vi "SCAPE-SpatialResolutionNumericalSimulation-4.vi"() -> ()   [LabVIEW 2024]
uses:
  <vilib>/Analysis/coordinate.llb/3D Cartesian Coordinate Rotation (Euler) (Scalar).vi
  <vilib>/Analysis/_algsub.llb/Real Vector Norm.vi
  <vilib>/Analysis/NI_AALPro.lvlib
  <vilib>/vision/NI_Vision_Development_Module.lvlib
panel:
  in  "r increment":dbl=2.0
  out "index":i32
  in  "iterataion":i32=1
  out "Array 2":dbl[][](array[numeric])=[[0.297159721790366, 0.6131743105327635, 1.1542088695697097]]
  out "x*y":dbl=2.94
  out "PSFxy":u16[][](graph)
  out "PSFxz":u16[][](graph)
  in  "y":dbl=0.7
  out "Image 3":T1(plugin-control)
  out "Image":T1(plugin-control)
  out "xy":u16[][](graph)
  out "zx":u16[][](graph)
  out "size(s) 3":i32[](array[numeric])=[256, 335, 256]
  out "size(s) 2":i32[](array[numeric])=[335, 256, 256]
  out "size(s)":i32[](array[numeric])=[110, 256, 256]
  in  "Angle (degrees)":dbl=45.0 format="%.2f"
  in  "perpendicular(T)/parallel(F)":bool=TRUE
  out "element":i32=127
  out "FWHMz":dbl=1.1542088695697097
  out "PSFz":u16[](graph)=[402, 405, 408, 411, 413, 415, 416, 417, 419, 420, 422, 424, 426, 429, 433, 437, 443, 450, 459, 468, 479, 493, 507, 524, 542, 563, 585, 610, 637, 666, 696, 730, 765, 802, 842, 883, 926, 970, 1017, 1065, 1114, 1164, 1215, 1267, 1320, 1372, 1423, 1475, 1528, 1579, 1629, 1677, 1725, 1771, 1814, 1855, 1895, 1933, 1966, 1997, 2026, 2054, 2076, 2095, 2114, 2127, 2139, 2149, 2155, 2161, 2165, 2167, 2169, 2171, 2174, 2177, 2181, 2189, 2199, 2215, 2236, 2260, 2296, 2339, 2389, 2450, 2526, 2613, 2710, 2831, 2966, 3116, 3289, 3485, 3699, 3935, 4205, 4496, 4807, 5160, 5541, 5947, 6384, 6863, 7372, 7909, 8493, 9109, 9760, 10451, 11182, 11941, 12740, 13591, 14473, 15375, 16329, 17325, 18356, 19398, 20489, 21616, 22778, 23953, 25153, 26390, 27662, 28941, 30221, 31535, 32879, 34233, 35557, 36903, 38273, 39669, 40991, 42317, 43664, 45034, 46319, 47585, 48860, 50137, 51344, 52506, 53661, 54778, 55867, 56881, 57839, 58771, 59697, 60509, 61237, 61944, 62648, 63212, 63707, 64160, 64583, 64893, 65139, 65318, 65421, 65478, 65463, 65328, 65141, 64938, 64646, 64221, 63759, 63289, 62709, 62051, 61334, 60597, 59778, 58919, 57976, 56989, 55982, 54953, 53810, 52645, 51486, 50309, 49035, 47748, 46476, 45186, 43856, 42496, 41153, 39811, 38472, 37087, 35723, 34386, 33076, 31715, 30387, 29093, 27832, 26560, 25311, 24097, 22924, 21771, 20633, 19529, 18480, 17459, 16452, 15494, 14580, 13703, 12846, 12040, 11270, 10536, 9845, 9188, 8562, 7980, 7437, 6921, 6434, 5997, 5586, 5199, 4848, 4529, 4234, 3962, 3724, 3504, 3305, 3133, 2979, 2840, 2720, 2620, 2531, 2452, 2391, 2339, 2295, 2260, 2233, 2211, 2195, 2185, 2177, 2171, 2168, 2166, 2164, 2162, 2160, 2157, 2152, 2144, 2135, 2125, 2110, 2092, 2073, 2053, 2026, 1996, 1966, 1933, 1896, 1856, 1815, 1772, 1727, 1680, 1631, 1581, 1531, 1479, 1427, 1374, 1324, 1271, 1219, 1168, 1117, 1069, 1021, 974, 929, 886, 845, 805, 768, 733, 699, 668, 638, 611, 587, 565, 543, 525, 509, 494, 481, 470, 460, 452, 445, 439, 434, 430, 427, 425, 424, 423, 423, 422, 421, 421, 420, 418, 416, 414, 412, 408, 404, 400, 394]
  in  "astigmatism (lambda)":dbl
  out "sum 2":dbl=26023.862010898454
  in  "image scan":bool=TRUE
  out "PSFy":u16[](graph)=[27, 29, 30, 31, 32, 34, 36, 38, 40, 42, 43, 45, 47, 49, 50, 52, 53, 54, 55, 55, 56, 56, 56, 57, 57, 57, 58, 59, 60, 62, 64, 67, 70, 75, 79, 85, 90, 96, 103, 110, 118, 126, 133, 141, 149, 157, 164, 172, 179, 186, 193, 200, 207, 214, 222, 230, 239, 249, 260, 272, 286, 301, 317, 334, 353, 372, 393, 414, 437, 459, 482, 505, 530, 555, 582, 611, 643, 679, 724, 778, 842, 919, 1023, 1150, 1298, 1484, 1714, 1993, 2323, 2712, 3166, 3708, 4340, 5047, 5837, 6774, 7815, 8952, 10197, 11603, 13125, 14754, 16516, 18402, 20401, 22510, 24722, 27017, 29388, 31833, 34323, 36849, 39374, 41890, 44389, 46860, 49225, 51501, 53677, 55731, 57617, 59333, 60845, 62163, 63287, 64182, 64762, 65141, 65324, 65206, 64801, 64179, 63367, 62266, 60951, 59430, 57726, 55852, 53833, 51644, 49349, 46980, 44547, 42027, 39492, 36956, 34429, 31931, 29480, 27085, 24774, 22555, 20437, 18426, 16528, 14742, 13104, 11595, 10191, 8891, 7768, 6749, 5822, 4993, 4295, 3684, 3145, 2686, 2301, 1982, 1716, 1493, 1308, 1165, 1052, 958, 880, 823, 776, 736, 702, 673, 645, 620, 594, 569, 545, 519, 494, 469, 444, 419, 395, 372, 350, 330, 311, 293, 277, 263, 249, 238, 227, 216, 208, 199, 191, 183, 175, 167, 160, 152, 145, 137, 130, 122, 115, 108, 101, 95, 89, 83, 78, 74, 70, 67, 65, 63, 61, 59, 59, 58, 58, 58, 57, 57, 57, 57, 56, 55, 54, 53, 52, 50, 49, 46, 44, 42, 40, 38, 36, 35, 33, 30, 29, 28]
  out "PSFx":u16[](graph)=[0, 0, 0, 1, 3, 4, 6, 8, 9, 10, 10, 10, 9, 7, 5, 3, 2, 1, 0, 0, 2, 4, 7, 10, 13, 16, 18, 19, 19, 17, 15, 12, 8, 5, 2, 0, 0, 2, 5, 10, 16, 22, 28, 33, 36, 37, 35, 32, 26, 19, 12, 6, 2, 1, 3, 9, 18, 30, 45, 59, 72, 82, 88, 88, 83, 72, 58, 41, 25, 11, 3, 3, 13, 32, 61, 98, 139, 180, 218, 248, 264, 266, 250, 219, 175, 125, 75, 36, 15, 22, 64, 144, 263, 417, 597, 790, 979, 1150, 1273, 1337, 1326, 1239, 1079, 861, 617, 390, 237, 226, 432, 949, 1839, 3184, 5045, 7468, 10473, 14056, 18182, 22784, 27765, 33003, 38349, 43637, 48719, 53369, 57442, 60787, 63274, 64806, 65324, 64806, 63274, 60787, 57442, 53369, 48719, 43512, 38239, 32910, 27688, 22722, 18135, 14023, 10452, 7458, 5043, 3189, 1849, 963, 463, 258, 270, 422, 646, 886, 1099, 1256, 1339, 1346, 1281, 1155, 985, 795, 601, 421, 267, 148, 68, 28, 21, 42, 82, 131, 180, 226, 255, 270, 267, 250, 220, 182, 140, 98, 62, 33, 14, 5, 5, 13, 27, 43, 60, 74, 84, 89, 89, 83, 73, 60, 45, 31, 19, 9, 3, 1, 3, 7, 13, 20, 27, 32, 36, 37, 37, 33, 28, 23, 16, 10, 6, 2, 1, 1, 2, 5, 8, 12, 15, 18, 19, 19, 18, 16, 13, 10, 7, 4, 2, 1, 0, 1, 2, 4, 6, 7, 9, 10, 10, 10, 9, 8, 6, 4, 3, 1, 0, 0]
  in  "r":dbl=12.77
  in  "w0y [um]":dbl=3.0
  in  "show entire PSFzy":bool=TRUE
  out "FWHMx":dbl=0.297159721790366
  out "pixel size xy":dbl=0.01640625
  out "appended array":string[](array[string])=["XLUMPLFL20X", "XLUMPLFL20X", "XLUMPLFL20X", "1.000000", "180.000000", "20.000000", "1.333000", "48.606626", "1.000000", "180.000000", "20.000000", "1.333000", "1.000000", "180.000000", "20.000000", "1.333000", "45.000000", "0.297160", "0.613174", "3.000000", "0.525000", "1.000000"]
  out "Obj name2":string="XLUMPLFL20X"
  out "Obj name3":string="XLUMPLFL20X"
  out "Obj name1":string="XLUMPLFL20X"
  out "FWHMy":dbl=0.6131743105327635
  in  "w0x [um]":dbl=3.0
  out "iz":i32=164
  in  "num of z":i32=110
  in  "z [um] step":dbl=0.05
  in  "wavelength [um]":dbl=0.525
  in  "Obj-3":i32
  in  "Obj-2":i32
  in  "Obj-1":i32
  in  "Array":T2(array[cluster])=[{"n"=1.333, "ft"=180.0, "mag"=20.0, "NA"=1.0, "name"="XLUMPLFL20X"}, {"n"=1.333, "ft"=180.0, "mag"=60.0, "NA"=1.2, "name"="UPLSAPO60XW"}, {"n"=1.0, "ft"=180.0, "mag"=40.0, "NA"=0.95, "name"="UPLSAPO40X"}, {"n"=1.0, "ft"=180.0, "mag"=20.0, "NA"=0.75, "name"="UPLSAPO20X"}, {"n"=1.0, "ft"=200.0, "mag"=10.0, "NA"=0.42, "name"="MPlApoHR10x"}, {"n"=1.0, "ft"=200.0, "mag"=5.0, "NA"=0.21, "name"="MPlApoHR5x"}, {"n"=1.0, "ft"=200.0, "mag"=10.0, "NA"=0.28, "name"="MPlApo10x"}, {"n"=1.0, "ft"=200.0, "mag"=5.0, "NA"=0.14, "name"="MPlApo5x"}, {"n"=1.0, "ft"=200.0, "mag"=20.0, "NA"=0.45, "name"="Nikon 20x"}, {"n"=1.4, "ft"=180.0, "mag"=30.0, "NA"=1.05, "name"="UPLSAPO30XSIR"}, {"n"=1.333, "ft"=200.0, "mag"=60.0, "NA"=1.27, "name"="MRD07650"}, {"n"=1.333, "ft"=200.0, "mag"=25.0, "NA"=1.1, "name"="CFI75 Apo"}, {"n"=1.333, "ft"=200.0, "mag"=40.0, "NA"=1.25, "name"="MRD77400"}]
  out "NAeff-max":dbl=1.0
  out "aperture radius1":dbl=9.0
  out "f1":dbl=11.997
  out "NA1":dbl=1.0
  out "theta1":dbl=48.60662639169028
  out "mag1":dbl=20.0
  out "ft1":dbl=180.0
  out "n1":dbl=1.333
  out "mag1-2":dbl=1.0000000000000002
  out "mag3":dbl=20.0
  out "ft3":dbl=180.0
  out "n2":dbl=1.333
  out "ft2":dbl=180.0
  out "mag2":dbl=20.0
  out "n3":dbl=1.333
  in  "color 3":T3={"color array"=[16711680, 16776960, 16711680, 16777215, 16776960, 16711680, 16448250, 16448250], "num of colors"=2, "max"=1.5200000000000005, "min"=1.0} {"min" step=0.01 format="%_2f"; "max" step=0.1 format="%_3f"}
  in  "autoscale 3":bool=TRUE
  out "Intensity Graph 3":dbl[][](graph)
  in  "autoscale":bool=TRUE
  in  "color 1":T3={"color array"=[0, 16711680, 16776960, 16448250, 65280, 16776960, 16711680, 16448250, 16448250], "num of colors"=4, "max"=1.1499999999999986, "min"=0.0} {"min" step=0.01 format="%_2f"; "max" step=0.1 format="%_3f"}
  out "sum":dbl=17.84765625
  out "theta2":dbl=48.60662639169028
  out "theta3":dbl=48.60662639169028
  out "NA2":dbl=1.0
  out "f3":dbl=11.997
  out "f2":dbl=11.997
  in  "oblique angle":dbl=45.0
  out "NA3":dbl=1.0
  in  "N of pixels":i32=256
  # "Note: this vi is valid only at n2 = n3."
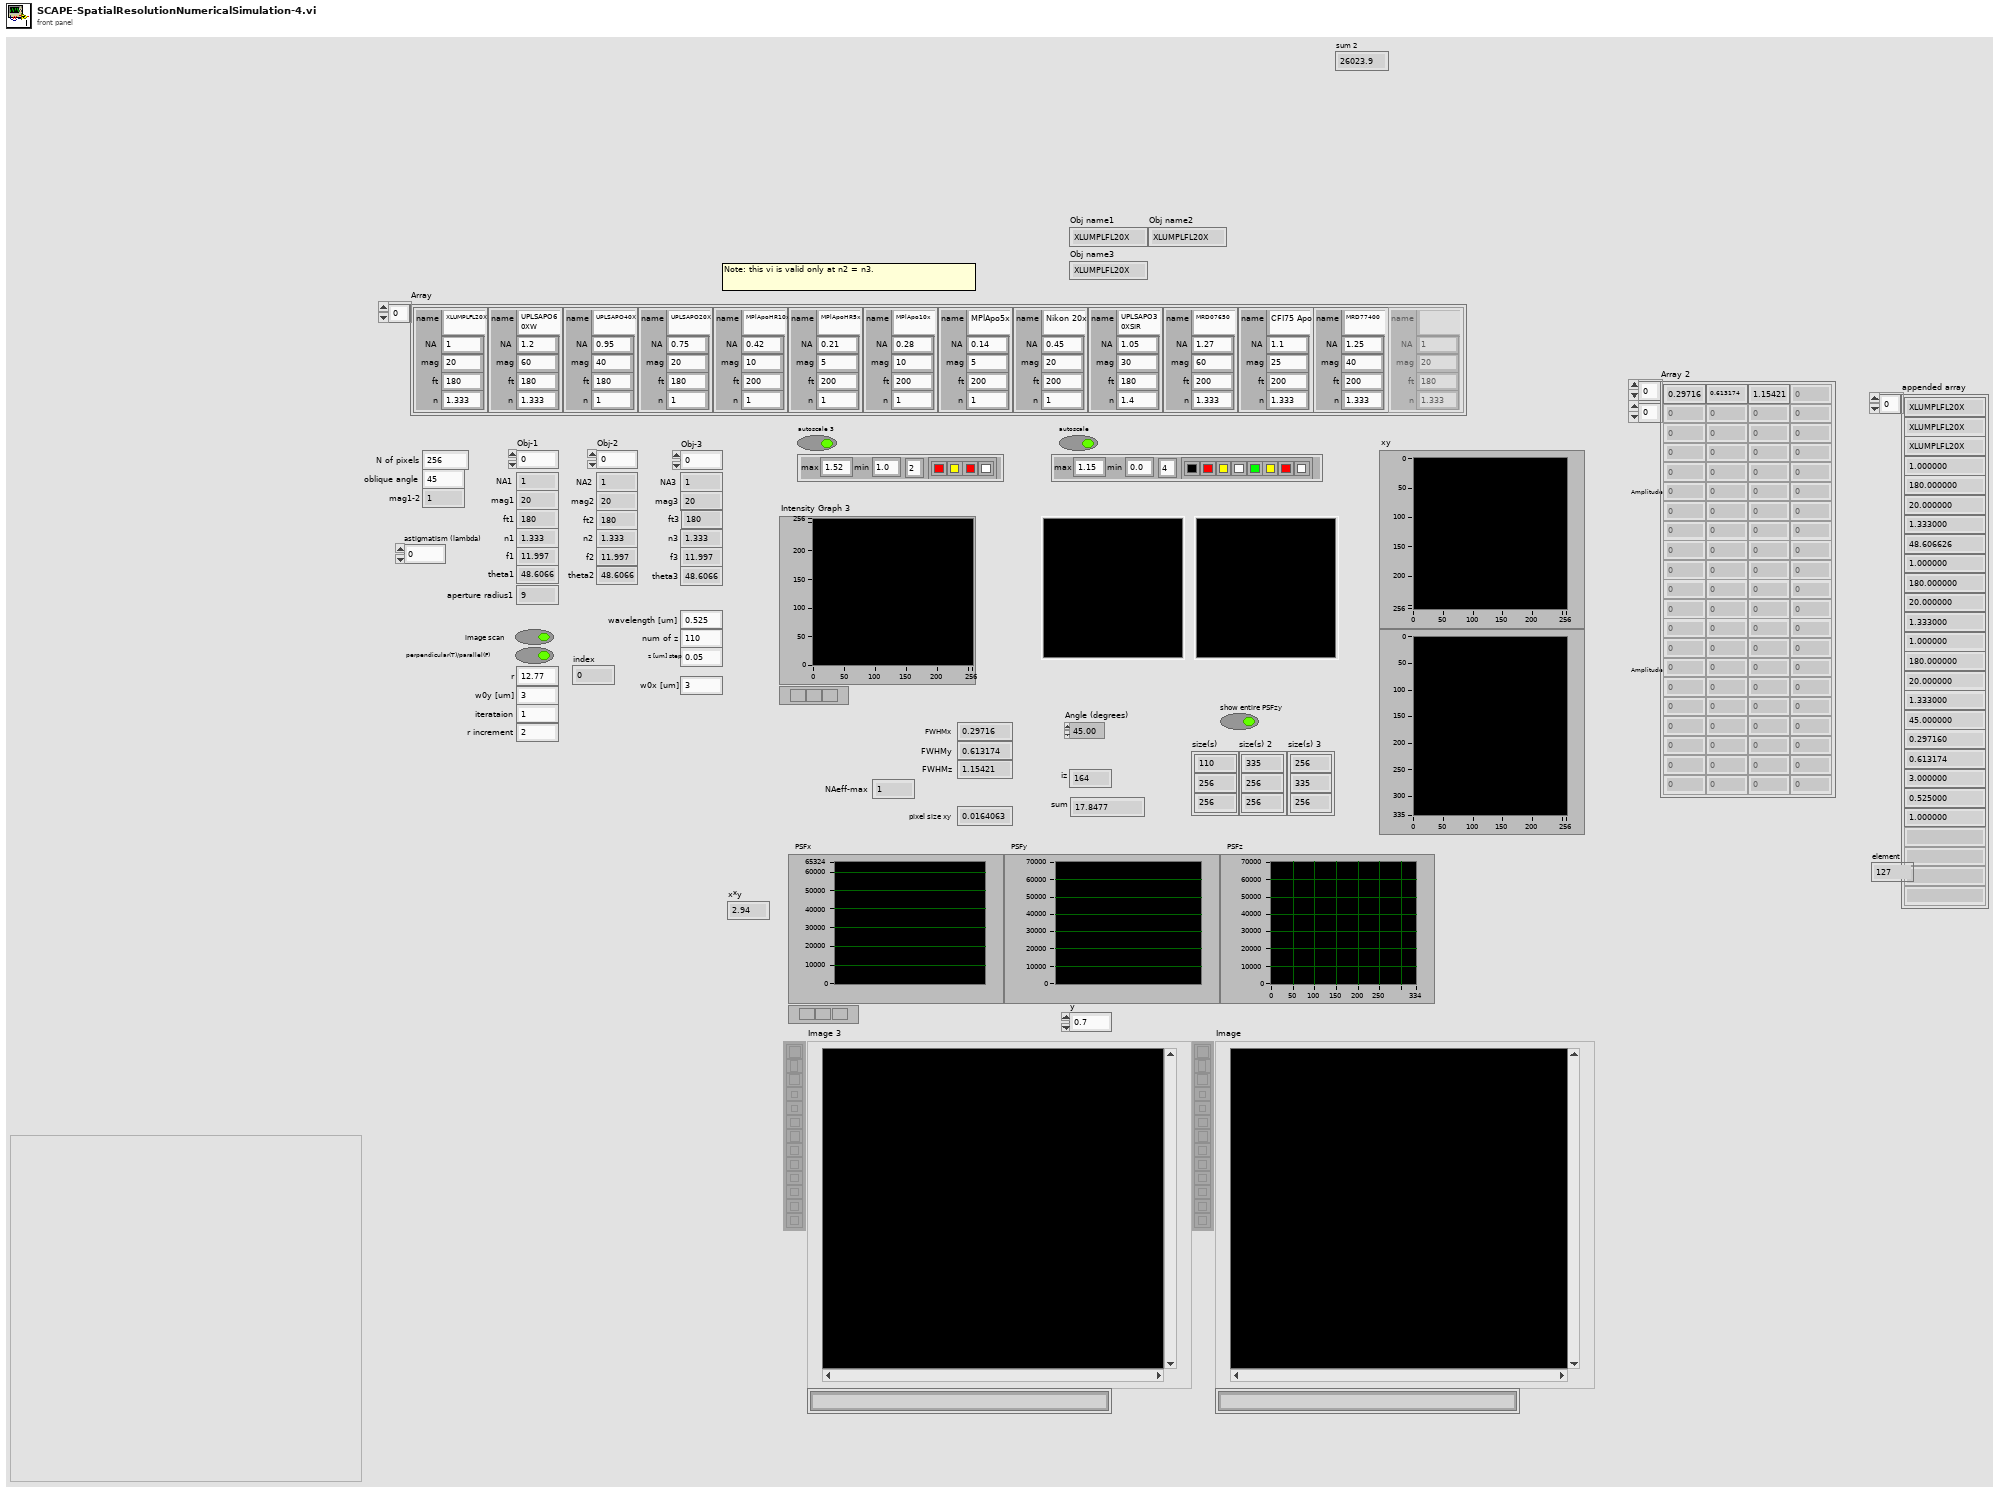
[diagram p1: front panel]
types:
  T1 = typedef "IMAQ Image.ctl" = refnum<image>
  T2 = cluster{"n":dbl, "ft":dbl, "mag":dbl, "NA":dbl, "name":string}[]
  T3 = cluster{"color array":u32[], "num of colors":i32, "max":dbl, "min":dbl}
  T4 = cluster{"n":dbl, "ft":dbl, "mag":dbl, "NA":dbl, "name":string}
  T5 = typedef "Image Type" = u32
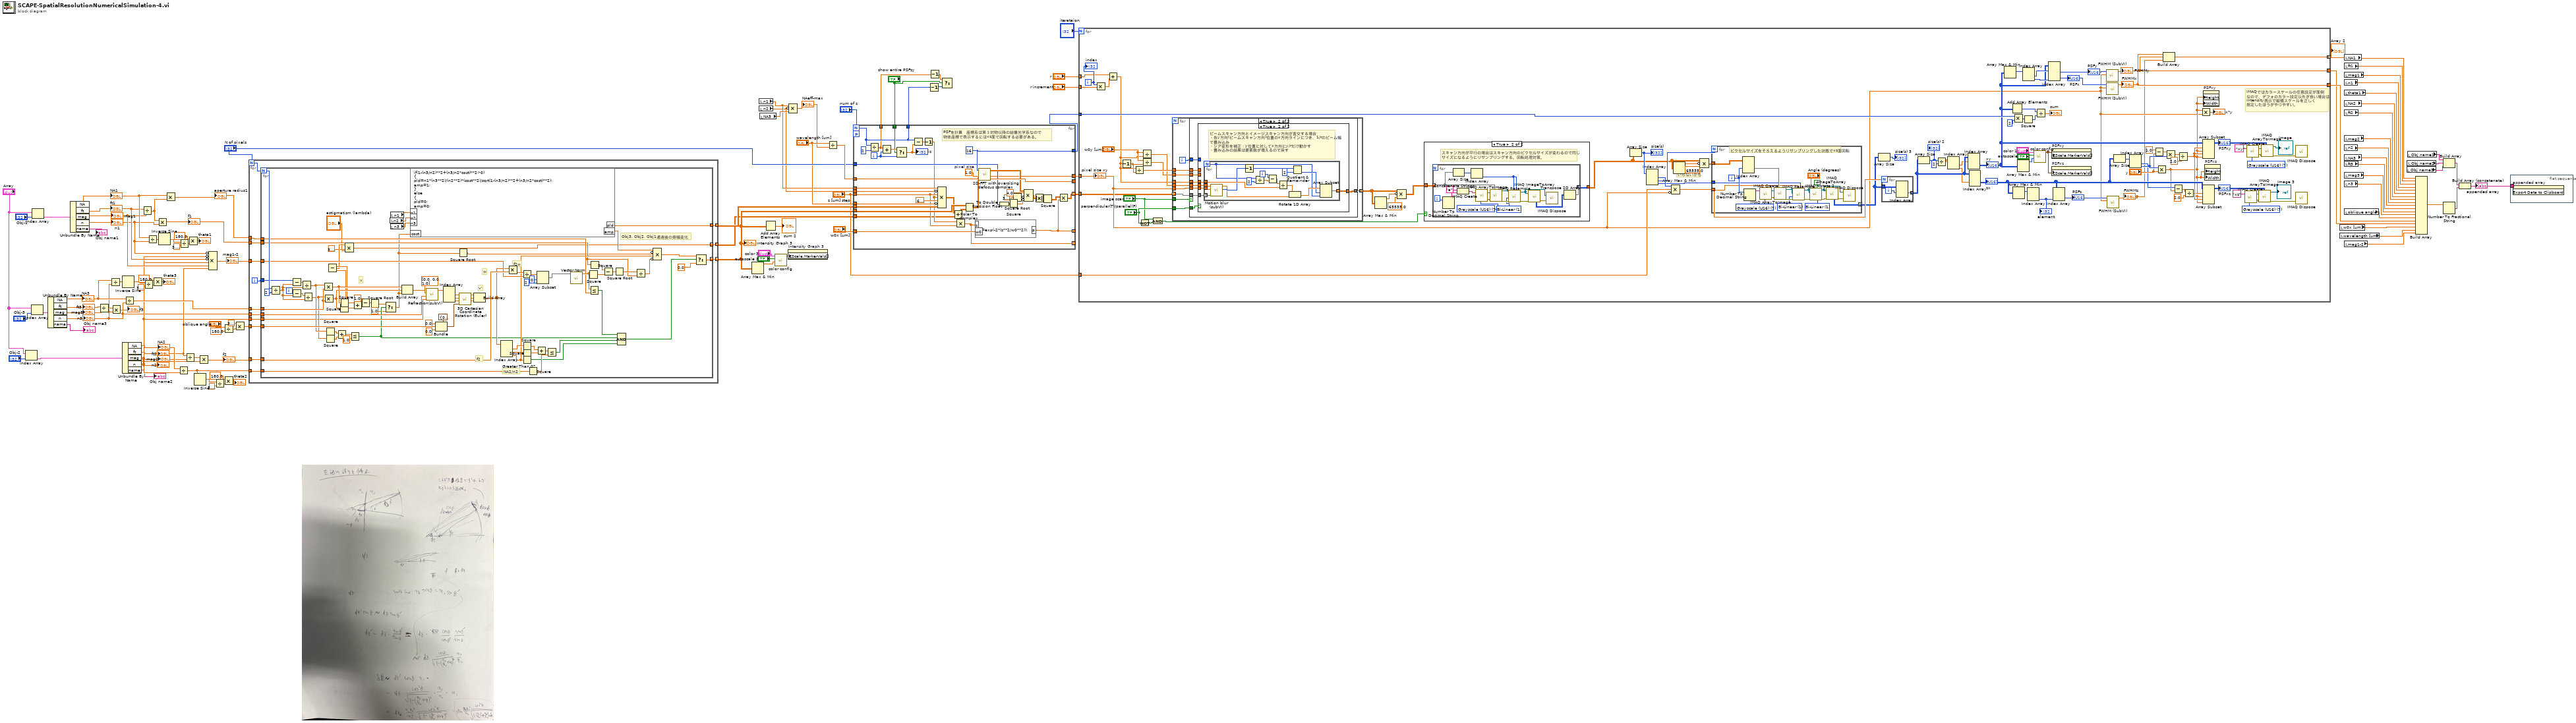
[diagram p0: block diagram]
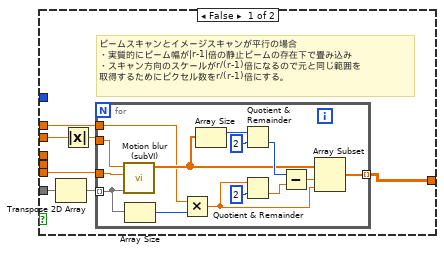
[diagram p4: hidden frame]
diagram:
  n1 = Index Array(array="Array", index="Obj-2") -> (element=w67:T4)
  n2 = Index Array(array="Array", index="Obj-3") -> (element=w68:T4)
  n3 = Index Array(array="Array", index="Obj-1") -> (element=w70:T4)
  n4 = Unbundle By Name(w68) -> ("NA"=w58:dbl, "ft"=w57:dbl, "mag"=w56:dbl, "n"=w55:dbl, "name"=→"Obj name3":string)
  "NA3" <- w58
  "n3" <- w55
  "mag3" <- w56
  "ft3" <- w57
  n5 = Unbundle By Name(w70) -> ("NA"=w66:dbl, "ft"=w65:dbl, "mag"=w64:dbl, "n"=w63:dbl, "name"=→"Obj name1":string)
  "NA1" <- w66
  "mag1" <- w64
  "ft1" <- w65
  "n1" <- w63
  n6 = Divide(x=w57, y=w56) -> (x/y=w88:dbl)
  n7 = Divide(x=w58, y=w55) -> (x/y=w78:dbl)
  n8 = Multiply(x=w88, y=w55) -> (x*y=→"f3":dbl)
  n9 = Unbundle By Name(w67) -> ("NA"=w62:dbl, "ft"=w61:dbl, "mag"=w60:dbl, "n"=w59:dbl, "name"=→"Obj name2":string)
  "NA2" <- w62
  "mag2" <- w60
  "ft2" <- w61
  "n2" <- w59
  n10 = Inverse Sine(1:w78) -> (0:w103:dbl)
  n11 = Divide(x=w58, y=w55) -> (x/y=w91:dbl)
  n12 = Divide(x=w65, y=w64) -> (x/y=w80:dbl)
  n13 = Divide(x=w103, y=3.141592653589793) -> (x/y=w102:dbl)
  n14 = Divide(x=w66, y=w63) -> (x/y=w77:dbl)
  n15 = Multiply(x=180.0, y=w102) -> (x*y=→"theta3":dbl)
  n16 = Multiply(x=w80, y=w63) -> (x*y=w81:dbl)
  "f1" <- w81
  n17 = Inverse Sine(1:w77) -> (0:w86:dbl)
  n18 = Multiply(x=w66, y=w80) -> (x*y=w79:dbl)
  "aperture radius1" <- w79
  n19 = Divide(x=w62, y=w59) -> (x/y=w76:dbl)
  n20 = Divide(x=w86, y=3.141592653589793) -> (x/y=w83:dbl)
  n21 = Divide(x=w61, y=w60) -> (x/y=w90:dbl)
  n22 = Multiply(x=180.0, y=w83) -> (x*y=→"theta1":dbl)
  n23 = Inverse Sine(1:w76) -> (0:w96:dbl)
  n24 = Multiply(x=w90, y=w59) -> (x*y=w89:dbl)
  "f2" <- w89
  n25 = Compound Arithmetic op=MULTIPLY(invert w63, invert w60, invert w65, w59, w64, w61) -> (w75:dbl)
  "mag1-2" <- w75
  n26 = Divide(x=w96, y=3.141592653589793) -> (x/y=w99:dbl)
  n27 = Divide(x="oblique angle", y=180.0) -> (x/y=w108:dbl)
  n28 = Multiply(x=180.0, y=w99) -> (x*y=→"theta2":dbl)
  n29 = Multiply(x=3.141592653589793, y=w108) -> (x*y=w106:dbl)
  n30 = for {
    N: "N of pixels" -> [w113]
    tunnel: w91 -> [w123]
    tunnel: w106 -> [w122]
    tunnel: w89 -> [w121]
    tunnel: w76 -> [w120]
    tunnel: [w119] -> w17 mode=indexing
    tunnel: w55 -> [w118]
    tunnel: w59 -> [w117]
    tunnel: w75 -> [w116]
    tunnel: w81 -> [w115]
    tunnel: w79 -> [w114]
    tunnel: [w112] -> w18 mode=indexing
    tunnel: [w111] -> w10 mode=indexing
    i -> [w124]
    n31 = for {
      N: w113 -> [w206]
      tunnel: w124 -> [w203]
      tunnel: w123 -> [w199]
      tunnel: w122 -> [w192]
      tunnel: w121 -> [w169]
      tunnel: w120 -> [w189]
      tunnel: [w174] -> w119 mode=indexing
      tunnel: w118 -> [w171]
      tunnel: w117 -> [w170]
      tunnel: w116 -> [w167]
      tunnel: w115 -> [w144]
      tunnel: w114 -> [w158]
      tunnel: [w136] -> w112 mode=indexing
      tunnel: [w127] -> w111 mode=indexing
      i -> [w204]
      # "n2 =! n3のときは不正確！　近似が成立しないので怪しい\nPSFxyは正しいがz方向の分布はおそらく間違っている"
      # "Obj3, Obj2, Obj1通過後の振幅変化"
      # "f2w"
      # "f2"
      # "NA2/n2"
      # "w"
      # "v"
      # "v'"
      n32 = Divide(x=w206, y=2) -> (x/y=w200:dbl)
      n33 = Subtract(x=w203, y=w200) -> (x-y=w202:dbl)
      n34 = Subtract(x=w204, y=w200) -> (x-y=w201:dbl)
      n35 = Divide(x=w202, y=w200) -> (x/y=w185:dbl)
      n36 = Divide(x=w201, y=w200) -> (x/y=w184:dbl)
      n37 = Multiply(x=w185, y=w199) -> (x*y=w153:dbl)
      n38 = Multiply(x=w184, y=w199) -> (x*y=w152:dbl)
      n39 = Square(x=w185) -> (x^2=w186:dbl)
      n40 = Square(x=w184) -> (x^2=w187:dbl)
      n41 = Add(x=w186, y=w187) -> (x+y=w188:dbl)
      n42 = Square(x=w152) -> (x^2=w129:dbl)
      n43 = Square(x=w153) -> (x^2=w130:dbl)
      n44 = Subtract(x=w130, y=w129) -> (x-y=w128:dbl)
      n45 = Compound Arithmetic op=MULTIPLY(w128, 3.141592653589793, "astigmatism (lambda)") -> (w127:dbl)
      n46 = Less Or Equal?(x=w188, y=1.0) -> (x <= y?=w135:bool)
      n47 = Add(x=w130, y=w129) -> (x+y=w197:dbl)
      n48 = Subtract(x=1.0, y=w197) -> (x-y=w196:dbl)
      n49 = Square Root(x=w196) -> (sqrt(x)=w140:dbl)
      n50 = Select(t=w140, s=w135, f=1.0) -> (s? t:f=w132:dbl)
      n51 = local read "n2"() -> (w138:dbl)
      n52 = local read "n1"() -> (w139:dbl)
      n53 = local read "n3"() -> (w137:dbl)
      n54 = Build Array(w153, w152, w132) -> (w143:dbl[])
      n55 = formula code="if(1-(n3/n2)**2+(n3/n2*cost)**2>0)\n{\npld=n1*(n3**2)/(n2**2)*(cost**2)/sqrt(1-(n3/n2)**2+(n3/n2*cost)**2);\namp=1;\n}\nelse\n{\npld=0;\namp=0;\n}"("n1"=w139, "n2"=w138, "n3"=w137, "cost"=w132) -> ("pld"=w136:dbl, "amp"=w133:dbl)
      n56 = call "Refraction(subVI).vi"("n2"=w170, "n1"=w171, "n"=dbl[] [0.0, 0.0, 1.0], "v1"=w143) -> ("v2"=w142:dbl[])  [unwired: 7 in]
      n57 = Bundle(cluster=cluster{"phi":dbl, "theta":dbl, "psi":dbl} {"phi"=0.0, "theta"=0.0, "psi"=0.0} ("Euler Angles"), "phi"=0.0, "theta"=w192, "psi"=0.0) -> (w173:cluster{"phi":dbl, "theta":dbl, "psi":dbl})
      n58 = Index Array(array=w142) -> (element #1=w151:dbl, element #2=w150:dbl, element #3=w149:dbl)  [unwired: 3 in]
      n59 = Square Root(x=w132) -> (sqrt(x)=w131:dbl)
      n60 = call-poly <vilib>:"3D Cartesian Coordinate Rotation (Euler).vi"("Euler Angles"=w173, "z"=w149, "y"=w150, "x"=w151) -> ("z out"=w180:dbl, "y out"=w181:dbl, "x out"=w182:dbl)  [unwired: 4 in, 1 out]
      n61 = Build Array(w182, w181, w180) -> (w148:dbl[])
      n62 = Index Array(array=w148) -> (element #1=w179:dbl, element #2=w178:dbl, element #3=w146:dbl)  [unwired: 3 in]
      n63 = Multiply(x=w148, y=w169) -> (x*y=w168:dbl[])
      n64 = Divide(x=w168, y=w167) -> (x/y=w166:dbl[])
      n65 = Square(x=w179) -> (x^2=w191:dbl)
      n66 = Square(x=w178) -> (x^2=w190:dbl)
      n67 = Greater Than 0?(x=w146) -> (x > 0?=w154:bool)
      n68 = Square(x=w189) -> (x^2=w177:dbl)
      n69 = Add(x=w191, y=w190) -> (x+y=w147:dbl)
      n70 = Array Subset(array=w166, index=0, length=2) -> (w163:dbl[])
      n71 = Less Or Equal?(x=w147, y=w177) -> (x <= y?=w155:bool)
      n72 = call-poly <vilib>:"Vector Norm.vi"("Input Vector"=w163) -> ("norm"=w159:dbl)  [unwired: 9 in, 1 out]
      n73 = Square(x=w159) -> (x^2=w162:dbl)
      n74 = Less Or Equal?(x=w159, y=w158) -> (x <= y?=w156:bool)
      n75 = Square(x=w144) -> (x^2=w161:dbl)
      n76 = Subtract(x=w161, y=w162) -> (x-y=w160:dbl)
      n77 = Square Root(x=w160) -> (sqrt(x)=w145:dbl)
      n78 = Compound Arithmetic op=AND(w156, w135, w155, w154) -> (w176:bool)
      n79 = Divide(x=w145, y=w144) -> (x/y=w141:dbl)
      n80 = Compound Arithmetic op=MULTIPLY(w133, invert w131, w146, invert w141) -> (w157:dbl)
      n81 = Select(t=w157, s=w176, f=0.0) -> (s? t:f=w174:dbl)
    }
  }
  "Intensity Graph 3" <- w17
  n82 = Array Max & Min(array=w17) -> (max value=w53:dbl)  [unwired: 3 out]
  n83 = local read "n1"() -> (w49:dbl)
  n84 = local read "n2"() -> (w48:dbl)
  n85 = local read "NA3"() -> (w74:dbl)
  n86 = Add Array Elements(numeric array=w17) -> (sum=→"sum 2":dbl)
  n87 = call "color config.vi"("max"=w53, "autoscale"="autoscale 3", "color 1"="color 3") -> ("Array"=w94:cluster{dbl, u32}[])  [unwired: 7 in, 1 out]
  n88 = property on="Intensity Graph 3" class="IntGraph (strict)"("ZScale.MarkerVals[]"=w94) -> ()  [unwired: 2 in, 2 out]
  n89 = Compound Arithmetic op=MULTIPLY(w49, invert w48, w74) -> (w46:dbl)
  "NAeff-max" <- w46
  n90 = Divide(x="wavelength [um]", y=w46) -> (x/y=w54:dbl)
  n91 = for {
    N: "num of z" -> [w214]
    tunnel: [w244] -> w95
    tunnel: [w243] -> _
    tunnel: w54 -> [w242]
    tunnel: w17 -> [w231]
    tunnel: "z [um] step" -> [w223]
    tunnel: w18 -> [w226]
    tunnel: "N of pixels" -> [w232]
    tunnel: [w221] -> _ mode=indexing
    tunnel: "wavelength [um]" -> [w230]
    workers-P: _ -> [_]
    tunnel: w49 -> [w228]
    tunnel: w48 -> [w227]
    tunnel: "w0x [um]" -> [w222]
    tunnel: [w207] -> _ mode=indexing
    tunnel: "show entire PSFzy" -> [w215]
    tunnel: [w214] -> w13
    tunnel: [w213] -> w12
    tunnel: w10 -> [w211]
    tunnel: [w209] -> w6 mode=indexing
    tunnel: [w210] -> w7
    i -> [w217]
    w244 = 16 ("oversize factor")
    w245 = 1.0  # pixel size
    # "PSFを計算　座標系は第３対物以降の結像光学系なので\n物体座標で表示するにはxz面で回転する必要がある。"
    n92 = Divide(x=w214, y=2) -> (x/y=w213:dbl)
    n93 = Add(x=w213, y=w217) -> (x+y=w216:dbl)
    n94 = Select(t=w216, s=w215, f=w217) -> (s? t:f=w218:dbl)
    "iz" <- w218
    n95 = Subtract(x=w214, y=w218) -> (x-y=w241:dbl)
    n96 = Decrement(x=w241) -> (x-1=w220:dbl)
    n97 = Compound Arithmetic op=MULTIPLY(w228, invert w227, w223, w220, 6.283185307179586, invert w230, w226) -> (w225:dbl[][])
    n98 = Add(x=w225, y=w211) -> (x+y=w212:dbl[][])
    n99 = Multiply(x=w220, y=w223) -> (x*y=w221:dbl)
    n100 = Polar To Complex(1:w212, 2:w231) -> (0:w224:cdb[][])
    n101 = formula code="P=exp(-2*(z**2/w0**2));"("z"=w221, "w0"=w222) -> ("P"=w207:dbl)
    n102 = call "2D-FFT with oversizing defocus complex.vi"("Array in"=w224, "lambda/NA"=w242, "pixel size"=w245, "oversize factor"=w244) -> ("Array"=w243:dbl[], "pixel size"=w210:dbl, "Array out"=w240:cdb[][])  [unwired: 5 in]
    n103 = To Double Precision Float(number=w232) -> (double precision float=w236:dbl)
    n104 = Square(x=w236) -> (x^2=w239:dbl)
    n105 = Square Root(x=3.141592653589793) -> (sqrt(x)=w238:dbl)
    n106 = Compound Arithmetic op=MULTIPLY(w240, 4.0 ("value"), invert w238, invert w239) -> (w237:cdb[][])
    n107 = Absolute Value(x=w237) -> (abs(x)=w235:dbl[][])
    n108 = Square(x=w235) -> (x^2=w208:dbl[][])
    n109 = Multiply(x=w208, y=w207) -> (x*y=w209:dbl[][])
  }
  n110 = Decrement(x=w13) -> (x-1=w15:i32)
  n111 = Decrement(x=w12) -> (x-1=w11:dbl)
  n112 = Select(t=w11, s="show entire PSFzy", f=w15) -> ()  [unwired: 1 out]
  n113 = for {
    N: "iterataion" -> [_]
    tunnel: w95 -> [w334]
    tunnel: "r" -> [w250]
    tunnel: "z [um] step" -> [w307]
    tunnel: w7 -> [w267]
    tunnel: w6 -> [w262]
    tunnel: [w257] -> w5
    tunnel: [w256] -> w4
    tunnel: [w254] -> w3 mode=indexing
    tunnel: "r increment" -> [w253]
    i -> [w252]
    w285 = T5 7 items=["Grayscale (U8)", "Grayscale (I16)", "Grayscale (SGL)", "Complex (CSG)", "RGB (U32)", "HSL (U32)", "RGB (U64)", "Grayscale (U16)"] ("Image Type")
    w296 = T5 7 items=["Grayscale (U8)", "Grayscale (I16)", "Grayscale (SGL)", "Complex (CSG)", "RGB (U32)", "HSL (U32)", "RGB (U64)", "Grayscale (U16)"] ("Image Type")
    # "いらないかも"
    # "IMAQではカラースケールの任意設定が面倒\nなので、デフォのカラー設定以外が良い場合は\nIntensity表示で縦横スケールを正しく\n指定したほうがやりやすい。"
    n114 = Multiply(x=w252, y=w253) -> (x*y=w251:dbl)
    n115 = Add(x=w250, y=w251) -> (x+y=w249:dbl)
    n116 = Decrement(x=w249) -> (x-1=w317:dbl)
    n117 = Divide(x=w249, y=w317) -> (x/y=w316:dbl)
    n118 = Not(x="perpendicular(T)/parallel(F)") -> (.not. x?=w313:bool)
    n119 = Divide(x="w0y [um]", y=w249) -> (x/y=w315:dbl)
    n120 = Divide(x="w0y [um]", y=w317) -> (x/y=w314:dbl)
    n121 = And(x="image scan", y=w313) -> (x .and. y?=w260:bool)
    n122 = for {
      tunnel: w249 -> [w390]
      tunnel: w316 -> [w389]
      tunnel: "image scan" -> [w388]
      tunnel: w267 -> [w387]
      tunnel: w315 -> [w386]
      tunnel: w262 -> [w385] mode=indexing
      tunnel: "perpendicular(T)/parallel(F)" -> [w384]
      tunnel: w314 -> [w383]
      tunnel: [w382] -> w261 mode=indexing
      i -> [w381]
      n123 = case shown="True" w388 {
        tunnel: w387 -> [_ w400]
        tunnel: w386 -> [_ w399]
        tunnel: [w391 w396] -> w382
        tunnel: w390 -> [_ w398]
        tunnel: w385 -> [w391 w397]
        tunnel: w384 -> [_ w395]
        tunnel: w383 -> [_ w394]
        tunnel: w389 -> [_ w393]
        tunnel: w381 -> [_ w392]
        frame False {
        }
        frame True {
          n124 = case shown="True" w395 {
            tunnel: w400 -> [w407 w426]
            tunnel: w399 -> [_ w425]
            tunnel: w398 -> [_ w424]
            tunnel: w397 -> [w406 w423]
            tunnel: [w402 w422] -> w396
            tunnel: w394 -> [w405 _]
            tunnel: w393 -> [w403 _]
            tunnel: w392 -> [_ _]
            frame False {
              # "ビームスキャンとイメージスキャンが平行の場合\n・実質的にビーム幅が|r-1|倍の静止ビームの存在下で畳み込み\n・スキャン方向のスケールがr/(r-1)倍になるので元と同じ範囲を\n取得するためにピクセル数をr/(r-1)倍にする。"
              n125 = Transpose 2D Array(2D array=w406) -> (transposed array=w404:dbl[][])
              n126 = Absolute Value(x=w405) -> (abs(x)=w401:dbl)
              n127 = for {
                tunnel: w404 -> [w414] mode=indexing
                tunnel: [w417] -> w402 mode=indexing
                tunnel: w407 -> [w421]
                tunnel: w401 -> [w420]
                tunnel: w403 -> [w409]
                n128 = call "Motion blur (subVI).vi"("Y"=w414, "pixel size [um]"=w421, "waist radius [um]"=w420) -> ("output"=w416:dbl[])  [unwired: 7 in, 1 out]
                n129 = Array Size(array=w414) -> (size(s)=w408:i32)
                n130 = Multiply(x=w409, y=w408) -> (x*y=w410:dbl)
                n131 = Array Size(array=w416) -> (size(s)=w415:i32)
                n132 = Quotient & Remainder(x=w415, y=2) -> (floor(x/y)=w418:i32)  [unwired: 1 out]
                n133 = Quotient & Remainder(x=w410, y=2) -> (floor(x/y)=w411:dbl)  [unwired: 1 out]
                n134 = Subtract(x=w418, y=w411) -> (x-y=w412:dbl)
                n135 = Array Subset(array=w416, index=w412, length=w410) -> (w417:dbl[])
              }
            }
            frame True {
              # "ビームスキャン方向とイメージスキャン方向が直交する場合\n・各y方向(ビームスキャン方向)位置のx方向ラインにつき、1/rのビーム幅\nで畳み込み\n・シア変形を補正：y位置に対してx方向にy/rだけ動かす\n・畳み込みの結果は要素数が増えるので戻す"
              n136 = for {
                N -> [w428]
                tunnel: w423 -> [w443] mode=indexing
                tunnel: [w427] -> w422 mode=indexing
                tunnel: w426 -> [w442]
                tunnel: w425 -> [w441]
                tunnel: w424 -> [w439]
                i -> [w433]
                n137 = call "Motion blur (subVI).vi"("Y"=w443, "pixel size [um]"=w442, "waist radius [um]"=w441) -> ("N"=w437:i32, "output"=w436:dbl[])  [unwired: 7 in]
                n138 = Decrement(x=w437) -> (x-1=w431:i32)
                n139 = Divide(x=w428, y=2) -> (x/y=w435:dbl)
                n140 = Subtract(x=w433, y=w435) -> (x-y=w434:dbl)
                n141 = Divide(x=w434, y=w439) -> (x/y=w438:dbl)
                n142 = Rotate 1D Array(1:w436, 2:w438) -> (0:w430:dbl[])
                n143 = Quotient & Remainder(x=w431, y=2) -> (floor(x/y)=w429:i32)  [unwired: 1 out]
                n144 = Array Subset(array=w430, index=w429, length=w428) -> (w427:dbl[])
              }
            }
          }
        }
      }
    }
    n145 = Array Max & Min(array=w261) -> (max value=w264:dbl)  [unwired: 3 out]
    n146 = Compound Arithmetic op=MULTIPLY(w261, invert w264, 65535.0 ("value")) -> (w259:dbl[][][])
    n147 = case shown="True" w260 {
      tunnel: w259 -> [w336 w338]
      tunnel: [w336 w337] -> w258
      frame False {
      }
      frame True {
        # "スキャン方向が平行の場合はスキャン方向のピクセルサイズが変わるので同じ\nサイズになるようにリサンプリングする。回転処理対策。"
        n148 = for {
          tunnel: w338 -> [w341] mode=indexing
          tunnel: [w342] -> w337 mode=indexing
          i -> [w343]
          w345 = u32 1 items=["Zero Order", "Bi-Linear", "Quadratic", "Cubic Spline"] ("Interpolation Type")
          w346 = T5 7 items=["Grayscale (U8)", "Grayscale (I16)", "Grayscale (SGL)", "Complex (CSG)", "RGB (U32)", "HSL (U32)", "RGB (U64)", "Grayscale (U16)"] ("Image Type")
          n149 = Number To Decimal String(number=w343) -> (decimal integer string=w351:string)  [unwired: 1 in]
          n150 = Array Size(array=w341) -> (size(s)=w340:i32[])
          n151 = Concatenate Strings("a" ("string"), w351) -> (w356:string)
          n152 = Index Array(array=w340) -> (element=w339:i32)  [unwired: 1 in]
          n153 = call "IMAQ Create"("Image Name"=w356, "Image Type"=w346) -> ("New Image"=w348:T1, "error out"=w350:errorcluster)  [unwired: 3 in]
          n154 = call "IMAQ ArrayToImage"("Image Pixels (U16)"=w341, "error in (no error)"=w350, "Image"=w348) -> ("error out"=w347:errorcluster, "Image Out"=w353:T1)  [unwired: 7 in]
          n155 = call "IMAQ Resample"("X Resolution"=w339, "Y Resolution"=w339, "error in (no error)"=w347, "Interpolation Type"=w345, "Image Dst"=w353, "Image Src"=w353) -> ("error out"=w352:errorcluster, "Image Dst Out"=w354:T1)  [unwired: 4 in]
          n156 = call "IMAQ ImageToArray"("error in (no error)"=w352, "Image"=w354) -> ("Image Pixels (U16)"=w355:u16[][], "error out"=w349:errorcluster)  [unwired: 2 in, 3 out]
          n157 = call "IMAQ Dispose"("Image"=w354, "error in (no error)"=w349) -> ()  [unwired: 4 in, 1 out]
          n158 = Transpose 2D Array(2D array=w355) -> (transposed array=w342:u16[][])
        }
      }
    }
    n159 = Array Size(array=w258) -> (size(s)=w310:i32[])
    "size(s)" <- w310
    n160 = Index Array(array=w310) -> (element #1=w308:i32, element #2=w309:i32, element #3=w306:i32)  [unwired: 3 in]
    n161 = Compound Arithmetic op=MULTIPLY(w308, w307, invert w267) -> (w305:dbl)
    n162 = Array Max & Min(array=w258) -> (max value=w248:dbl)  [unwired: 3 out]
    n163 = Compound Arithmetic op=MULTIPLY(w258, invert w248, 65535.0 ("value")) -> (w246:dbl[][][])
    n164 = for {
      N: w309 -> [_]
      tunnel: [w370] -> w303 mode=indexing
      tunnel: w306 -> [w362]
      tunnel: w305 -> [w363]
      tunnel: w246 -> [w360]
      i -> [w372]
      w364 = u32 1 items=["Zero Order", "Bi-Linear", "Quadratic", "Cubic Spline"] ("Interpolation Type")
      w368 = T5 7 items=["Grayscale (U8)", "Grayscale (I16)", "Grayscale (SGL)", "Complex (CSG)", "RGB (U32)", "HSL (U32)", "RGB (U64)", "Grayscale (U16)"] ("Image Type")
      w374 = 1 items=["Zero Order", "Bi-Linear"] ("Interpolation Type")
      # "ピクセルサイズをそろえるようリサンプリングした状態でxz面回転"
      n165 = Index Array(array=w360, index (dim 1)=w372) -> (element=w371:dbl[][])  [unwired: 2 in]
      n166 = Number To Decimal String(number=w372) -> (decimal integer string=w380:string)  [unwired: 1 in]
      n167 = call "IMAQ Create"("Image Name"=w380, "Image Type"=w368) -> ("New Image"=w376:T1, "error out"=w379:errorcluster)  [unwired: 3 in]
      n168 = call "IMAQ ArrayToImage"("Image Pixels (U16)"=w371, "error in (no error)"=w379, "Image"=w376) -> ("error out"=w366:errorcluster, "Image Out"=w361:T1)  [unwired: 7 in]
      n169 = call "IMAQ Resample"("X Resolution"=w362, "Y Resolution"=w363, "error in (no error)"=w366, "Interpolation Type"=w364, "Image Dst"=w361, "Image Src"=w361) -> ("error out"=w365:errorcluster, "Image Dst Out"=w367:T1)  [unwired: 4 in]
      n170 = call "IMAQ Rotate 2"("Interpolation Type"=w374, "Maintain Size"=TRUE, "error in (no error)"=w365, "Angle (degrees)"="Angle (degrees)", "Image Dst"=w367, "Image Src"=w367) -> ("error out"=w378:errorcluster, "Image Dst Out"=w375:T1)  [unwired: 4 in]
      n171 = call "IMAQ ImageToArray"("error in (no error)"=w378, "Image"=w375) -> ("Image Pixels (U16)"=w370:u16[][], "error out"=w377:errorcluster)  [unwired: 2 in, 3 out]
      n172 = call "IMAQ Dispose"("Image"=w375, "error in (no error)"=w377) -> ()  [unwired: 4 in, 1 out]
    }
    n173 = Array Size(array=w303) -> (size(s)=→"size(s) 3":i32[])
    n174 = for {
      N: w305 -> [_]
      tunnel: w303 -> [w359]
      tunnel: [w358] -> w302 mode=indexing
      i -> [w357]
      n175 = Index Array(array=w359, index (dim 1)=w357) -> (element=w358:u16[][])  [unwired: 2 in]
    }
    n176 = Array Size(array=w302) -> (size(s)=w300:i32[])
    "size(s) 2" <- w300
    n177 = Divide(x=w300, y=2) -> (x/y=w299:dbl[])
    n178 = Index Array(array=w299) -> (element #1=w298:dbl, element #2=w297:dbl)  [unwired: 2 in]
    n179 = Index Array(array=w302, index (dim 0)=w298) -> (element=w284:u16[][])  [unwired: 2 in]
    "xy" <- w284
    n180 = Index Array(array=w302, index (dim 1)=w297) -> (element=w283:u16[][])  [unwired: 2 in]
    "zx" <- w283
    n181 = Array Max & Min(array=w284) -> (max index (indices)=w326:i32[])  [unwired: 3 out]
    n182 = Add Array Elements(numeric array=w284) -> (sum=w335:u16)
    n183 = Multiply(x=w334, y=2) -> (x*y=w331:i32)
    n184 = Array Max & Min(array=w283) -> (max index (indices)=w321:i32[])  [unwired: 3 out]
    n185 = Array Max & Min(array=w284) -> (max value=w327:u16)  [unwired: 3 out]
    n186 = Index Array(array=w326) -> (element #1=w322:i32, element #2=w323:i32)  [unwired: 2 in]
    n187 = Square(x=w331) -> (x^2=w333:i32)
    n188 = Index Array(array=w321) -> (element #2=w320:i32)  [unwired: 2 in, 1 out]
    "element" <- w320
    n189 = call "color config.vi"("max"=w327, "autoscale"="autoscale", "color 1"="color 1") -> ("Array"=w265:cluster{dbl, u32}[])  [unwired: 7 in, 1 out]
    n190 = Divide(x=w335, y=w333) -> (x/y=→"sum":dbl)
    n191 = Index Array(array=w284, index (row) #1=w322, index (col) #2=w323) -> (element #1=w324:u16[], element #2=w325:u16[])  [unwired: 2 in]
    "PSFx" <- w325
    "PSFy" <- w324
    n192 = property on="PSFxy" class="IntGraph (strict)"("ZScale.MarkerVals[]"=w265) -> ()  [unwired: 2 in, 2 out]
    n193 = property on="PSFxz" class="IntGraph (strict)"("ZScale.MarkerVals[]"=w265) -> ()  [unwired: 2 in, 2 out]
    n194 = Index Array(array=w283, index (col)=w320) -> (element=w319:u16[])  [unwired: 1 in]
    "PSFz" <- w319
    n195 = call "FWHM (SubVI).vi"("Numeric in"=w267, "horizontalDBL"=w324) -> ("Numeric out"=w256:dbl)  [unwired: 9 in]
    "FWHMy" <- w256
    n196 = call "FWHM (SubVI).vi"("Numeric in"=w267, "horizontalDBL"=w325) -> ("Numeric out"=w257:dbl)  [unwired: 9 in]
    "FWHMx" <- w257
    n197 = call "FWHM (SubVI).vi"("Numeric in"=w267, "horizontalDBL"=w319) -> ("Numeric out"=w255:dbl)  [unwired: 9 in]
    "FWHMz" <- w255
    n198 = Array Size(array=w283) -> (size(s)=w280:i32[])
    n199 = Index Array(array=w280) -> (element #1=w274:i32, element #2=w277:i32)  [unwired: 2 in]
    n200 = Subtract(x=1.0, y="y") -> (x-y=w279:dbl)
    n201 = Multiply(x=w277, y="y") -> (x*y=w268:dbl)
    n202 = Build Array(w257, w256, w255) -> (w254:dbl[])
    n203 = Multiply(x=w279, y=w277) -> (x*y=w278:dbl)
    n204 = Subtract(x=w274, y=w268) -> (x-y=w272:dbl)
    n205 = Divide(x=w278, y=2.0) -> (x/y=w275:dbl)
    n206 = Divide(x=w272, y=2.0) -> (x/y=w271:dbl)
    n207 = Multiply(x=w268, y=w267) -> (x*y=→"x*y":dbl)
    n208 = Array Subset(array=w284, index (row)=w275, length (row)=w268, index (col)=w275, length (col)=w268) -> (w269:u16[][])
    "PSFxy" <- w269
    n209 = Array Subset(array=w283, index (row)=w271, length (row)=w268, index (col)=w275, length (col)=w268) -> (w270:u16[][])
    "PSFxz" <- w270
    n210 = property on="PSFxy" class="IntGraph (strict)"("Height"=w268, "Width"=w268) -> ()  [unwired: 2 in, 2 out]
    n211 = property on="PSFxz" class="IntGraph (strict)"("Height"=w268, "Width"=w268) -> ()  [unwired: 2 in, 2 out]
    n212 = call "IMAQ Create"("Image Name"="xz", "Image Type"=w285) -> ("New Image"=w289:T1, "error out"=w286:errorcluster)  [unwired: 3 in]
    n213 = call "IMAQ Create"("Image Name"="xy", "Image Type"=w296) -> ("New Image"=w292:T1, "error out"=w295:errorcluster)  [unwired: 3 in]
    n214 = call "IMAQ ArrayToImage"("Image Pixels (U16)"=w270, "error in (no error)"=w286, "Image"=w289) -> ("error out"=w288:errorcluster, "Image Out"=→"Image 3":T1)  [unwired: 7 in]
    n215 = call "IMAQ ArrayToImage"("Image Pixels (U16)"=w269, "error in (no error)"=w295, "Image"=w292) -> ("error out"=w293:errorcluster, "Image Out"=→"Image":T1)  [unwired: 7 in]
    n216 = call "IMAQ Dispose"("error in (no error)"=w288) -> ()  [unwired: 5 in, 1 out]
    n217 = call "IMAQ Dispose"("error in (no error)"=w293) -> ()  [unwired: 5 in, 1 out]
    "pixel size xy" <- w267
    "index" <- w252
  }
  "Array 2" <- w3
  n218 = local read "w0x [um]"() -> (w21:dbl)
  n219 = local read "wavelength [um]"() -> (w20:dbl)
  n220 = local read "NA1"() -> (w29:dbl)
  n221 = local read "ft1"() -> (w30:dbl)
  n222 = local read "mag1"() -> (w31:dbl)
  n223 = local read "n1"() -> (w32:dbl)
  n224 = local read "theta1"() -> (w33:dbl)
  n225 = local read "NA2"() -> (w34:dbl)
  n226 = local read "ft2"() -> (w35:dbl)
  n227 = local read "mag2"() -> (w36:dbl)
  n228 = local read "n2"() -> (w37:dbl)
  n229 = local read "NA3"() -> (w38:dbl)
  n230 = local read "ft3"() -> (w39:dbl)
  n231 = local read "mag3"() -> (w40:dbl)
  n232 = local read "n3"() -> (w41:dbl)
  n233 = local read "oblique angle"() -> (w45:dbl)
  n234 = local read "mag1-2"() -> (w19:dbl)
  n235 = local read "Obj name3"() -> (w26:string)
  n236 = local read "Obj name2"() -> (w27:string)
  n237 = local read "Obj name1"() -> (w28:string)
  n238 = Build Array(w29, w30, w31, w32, w33, w34, w35, w36, w37, w38, w39, w40, w41, w45, w5, w4, w21, w20, w19) -> (w25:dbl[])
  n239 = Build Array(w28, w27, w26) -> (w24:string[])
  n240 = Number To Fractional String(number=w25) -> (F-format string=w23:string[])  [unwired: 3 in]
  n241 = Build Array (concatenate)(w24, w23) -> (w22:string[])
  "appended array" <- w22
  n242 = flat-sequence {
    tunnel: w22 -> [_]
    frame #0 {
      n243 = invoke on="appended array" class="Arr (strict)" method="Export Data to Clipboard"() -> ()  [unwired: 3 in, 3 out]
    }
  }
